vi "Main.vi"() -> ()   [LabVIEW 2020] (continued)
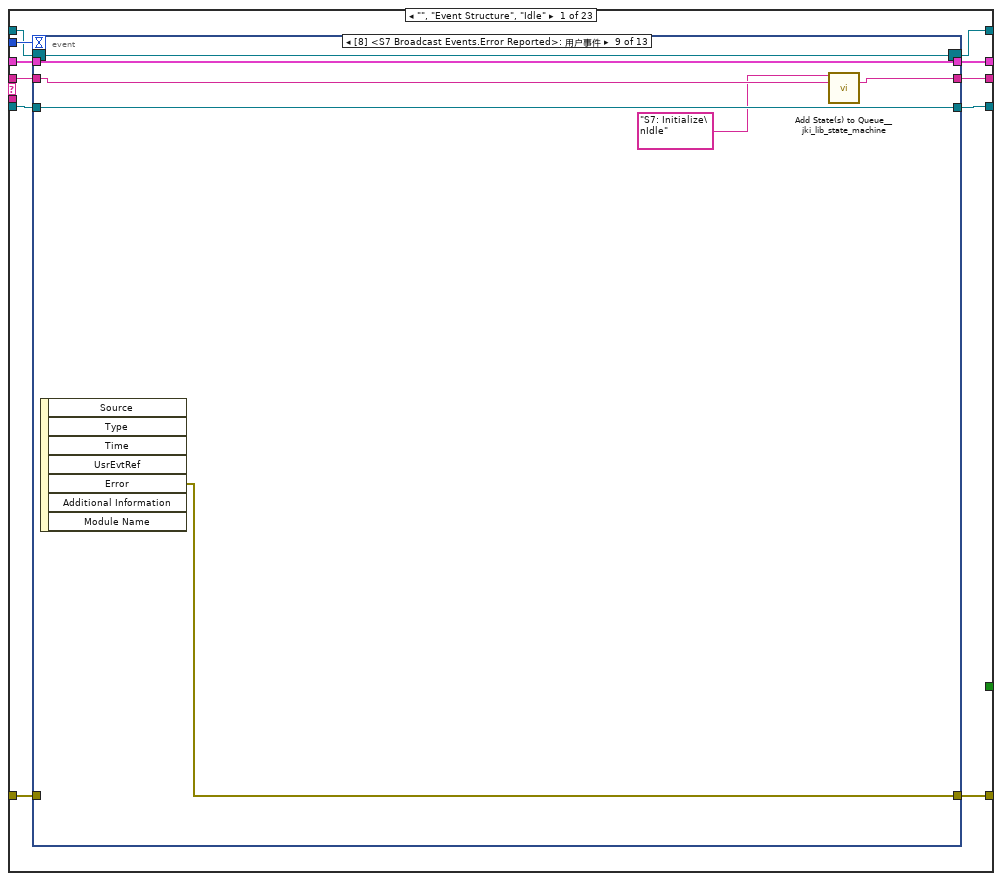
[diagram p2: hidden frame]
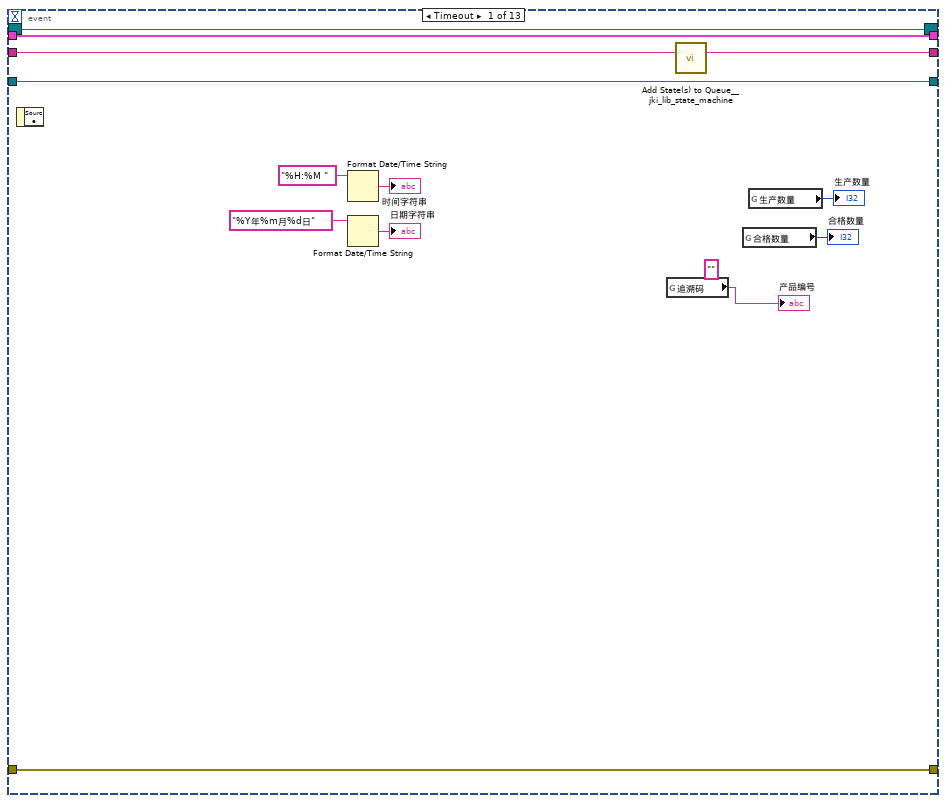
[diagram p3: hidden frame]
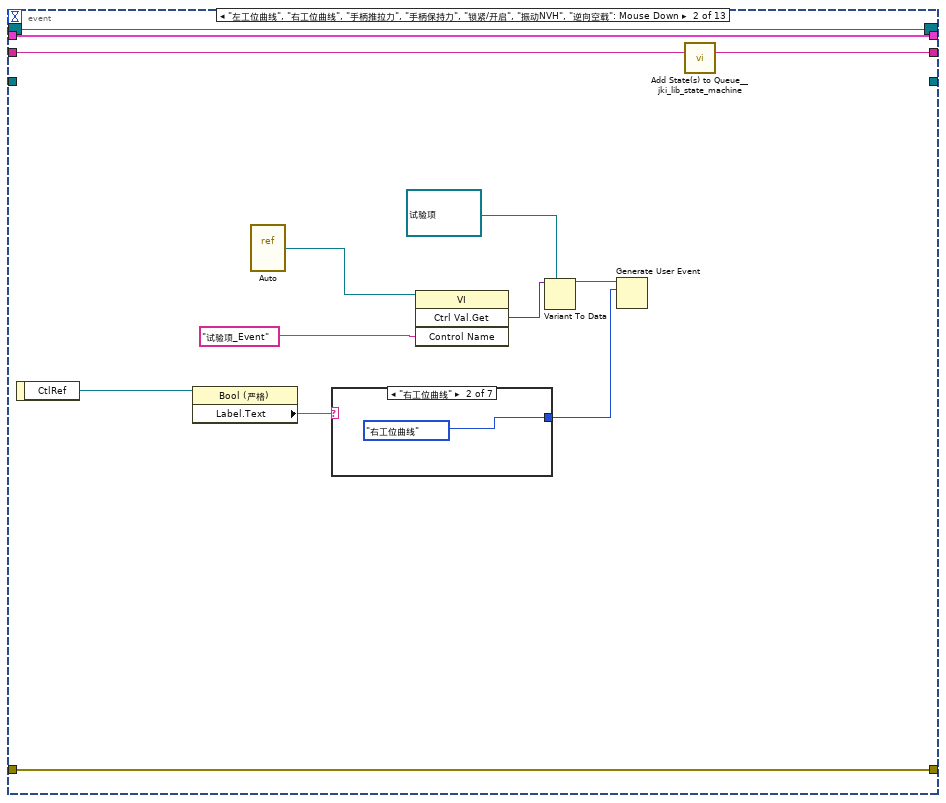
[diagram p4: hidden frame]
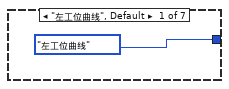
[diagram p5: hidden frame]
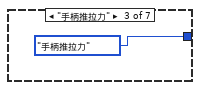
[diagram p6: hidden frame]
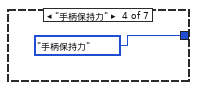
[diagram p7: hidden frame]
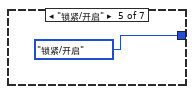
[diagram p8: hidden frame]
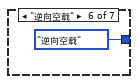
[diagram p9: hidden frame]
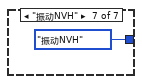
[diagram p10: hidden frame]
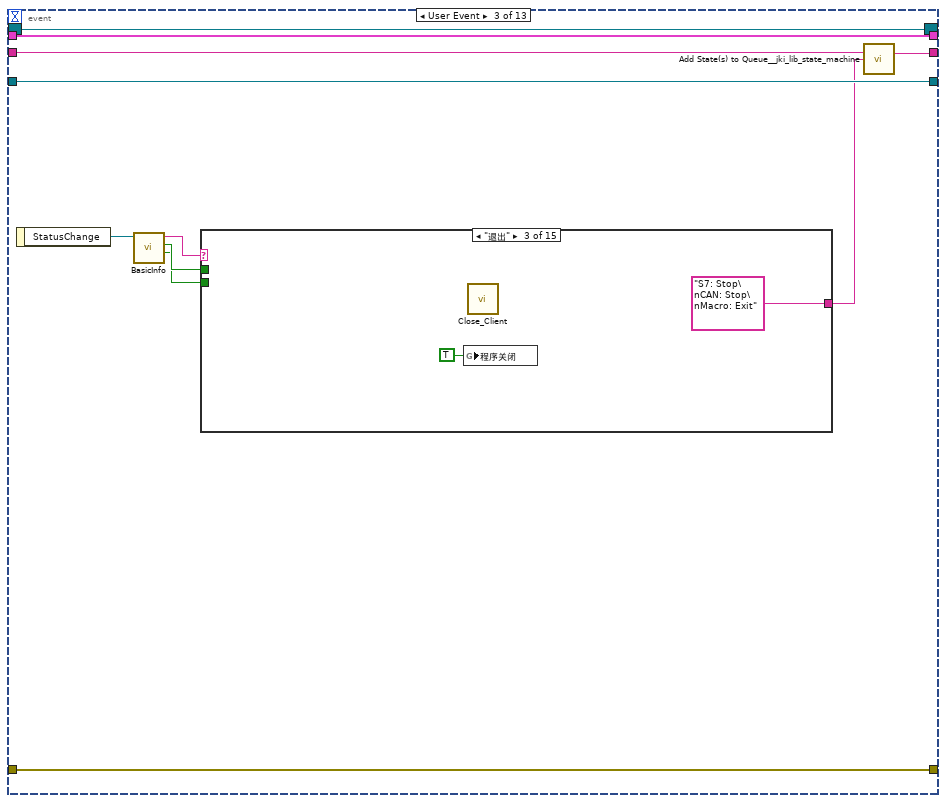
[diagram p11: hidden frame]
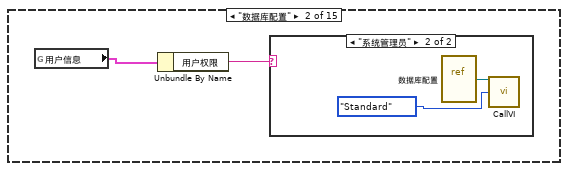
[diagram p13: hidden frame]
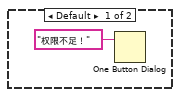
[diagram p14: hidden frame]
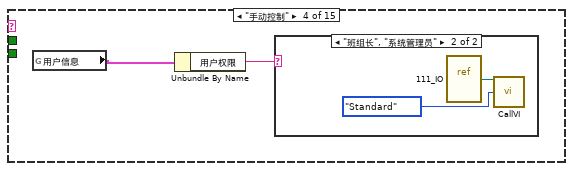
[diagram p15: hidden frame]
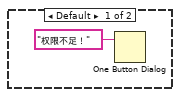
[diagram p16: hidden frame]
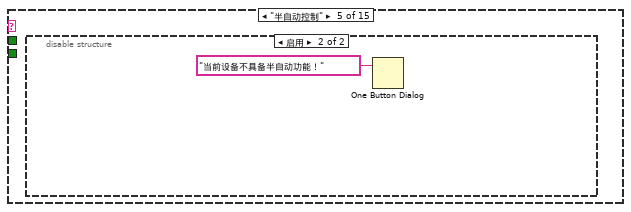
[diagram p17: hidden frame]
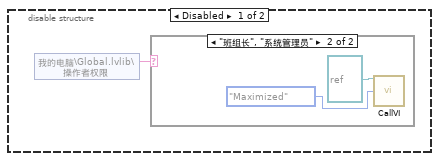
[diagram p18: hidden frame]
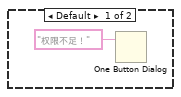
[diagram p19: hidden frame]
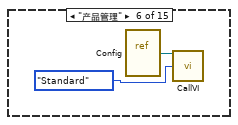
[diagram p20: hidden frame]
            n115 = call "CallVI.vi"("VI引用"=w195, "状态"=T6."Standard") -> ()  [unwired: 11 in, 3 out]
            n116 = call <vilib>:"Add State(s) to Queue__jki_lib_state_machine.vi"("State(s) in (\"\")"=w197) -> ("States Out"=w198:string)  [unwired: 14 in]
          }
          event Panel Close? {
            n117 = event-data() -> ()  [unwired: 1 in, 1 out]
            n118 = global write "Global.vi" "程序关闭"(TRUE ("程序关闭")) -> ()
            n119 = call <vilib>:"Add State(s) to Queue__jki_lib_state_machine.vi"("State(s) in Front (\"\")"="S7: Stop\nMacro: Exit", "State(s) in (\"\")"=w207) -> ("States Out"=w206:string)  [unwired: 13 in]
            n120 = event-data("Discard?"=TRUE) -> ()  [unwired: 1 in, 1 out]
          }
          event "产品更换": Value Change {
            n121 = event-data() -> ("NewVal"=w212:refnum<vi>)  [unwired: 1 in, 5 out]
            n122 = stacked-sequence {
              tunnel: w212 -> [w222 _]
              tunnel: [_ "Idle" ("State(s) in Front (\"\")")] -> w208
              frame #0 {
                n123 = disable-structure shown="禁用" {
                  disable-tunnel: w222 -> [w224 _]
                  frame Disabled {
                    n124 = control-ref of="子面板"() -> (w223:refnum<vi>)
                    n125 = call "Call_SubPanal.vi"("VI引用句柄"=w224, "SubPnl引用句柄"=w223) -> ()  [unwired: 9 in, 1 out]
                  }
                  frame Enabled {
                  }
                }
                n126 = vi-ref "Auto.vi"() -> (w216:refnum<vi>)
                n127 = global read "Global.vi" "产品型号"() -> (w215:string)
                n128 = invoke class="VI" method="Ctrl Val.Get"(reference=w216, "Control Name"="标尺_Event" ("控件名")) -> ("Get Control Value Variant"=w221:variant)  [unwired: 2 in, 3 out]
                n129 = Variant To Data(type=refnum<user-event> refnum ("标尺_Event"), Variant=w221) -> (data=w218:refnum<user-event>, error out=w217:errorcluster)  [unwired: 1 in]
                n130 = Generate User Event(user event=w218, event data cluster=w215, error in=w217) -> ()  [unwired: 1 in, 2 out]
                n131 = local write "产品型号"(w215) -> ()
              }
              frame #1 {
                n132 = control-ref of="锁紧/开启"() -> (w226:refnum<vi>)
                n133 = control-ref of="手柄保持力"() -> (w227:refnum<vi>)
                n134 = control-ref of="左工位曲线"() -> (w228:refnum<vi>)
                n135 = control-ref of="右工位曲线"() -> (w229:refnum<vi>)
                n136 = control-ref of="手柄推拉力"() -> (w230:refnum<vi>)
                n137 = global read "Global.vi" "试验项目"() -> (w233:bool[])
                n138 = Build Array(w228, w229, w230, w227, w226) -> (w232:refnum<vi>[])
                n139 = for {
                  tunnel: w232 -> [w237] mode=indexing
                  tunnel: w233 -> [w238] mode=indexing
                  shift-right: [w234] -> _
                  shift-left: 2000 -> [w235]
                  i -> [w236]
                  n140 = case shown="真" w238 {
                    tunnel: w237 -> [w239 w247]
                    tunnel: w236 -> [_ _]
                    tunnel: w235 -> [w241 w244]
                    tunnel: [w241 w242] -> w234
                    frame False {
                      n141 = property class="Bool (严格)"(reference=w239, "Top"=2000) -> ()  [unwired: 1 in, 2 out]
                    }
                    frame True {
                      n142 = Add(x=w244, y=180) -> (x+y=w242:i32)
                      n143 = Bundle(w242, 1230) -> (w245:cluster{i32, i32})  [unwired: 1 in]
                      n144 = property class="Bool (严格)"(reference=w247, "Position"=w245) -> ()  [unwired: 1 in, 2 out]
                    }
                  }
                }
              }
            }
            n145 = call <vilib>:"Add State(s) to Queue__jki_lib_state_machine.vi"("State(s) in Front (\"\")"=w208, "State(s) in (\"\")"=w210) -> ("States Out"=w209:string)  [unwired: 13 in]
          }
          event "Andon": Value Change {
            n146 = event-data() -> ("NewVal"=w252:enum32{"未选择", "缺料报警", "质量报警", "故障报警"})  [unwired: 1 in]
            n147 = case shown="\"未选择\", 默认" w252 {
              tunnel: [enum16{"设备离线", "设备正常", "设备缺料", "设备故障", "质量报警"}."设备正常" ("设备状态") enum16{"设备离线", "设备正常", "设备缺料", "设备故障", "质量报警"}."设备缺料" ("设备状态") enum16{"设备离线", "设备正常", "设备缺料", "设备故障", "质量报警"}."质量报警" ("设备状态") enum16{"设备离线", "设备正常", "设备缺料", "设备故障", "质量报警"}."设备故障" ("设备状态")] -> w250
              frame "未选择", Default {
              }
              frame "缺料报警" {
              }
              frame "质量报警" {
              }
              frame "故障报警" {
              }
            }
            n148 = local read "userName"() -> (w249:string)
            n149 = Bundle By Name(cluster=T7 {"设备名称"="调节机构检测", "操作人员"="", "设备状态"=enum."设备离线", "附加信息"=""} ("设备信息"), "操作人员"=w249, "设备状态"=w250) -> (w248:T7)
            n150 = call "Change_Client.vi"("设备信息"=w248) -> ()  [unwired: 10 in, 1 out]
          }
        }
      }
      frame "---------- Core ----------" {
        n151 = call <vilib>:"Add State(s) to Queue__jki_lib_state_machine.vi"("State(s) in (\"\")"=w266) -> ("States Out"=w265:string)  [unwired: 14 in]
      }
      frame Default {
        w278 = 42 items=["No error", "Argument error", "Memory is full", "Out of zone", "End of file", "File already open", "Generic file I/O error", "File not found", "File permission error", "Disk is full", "Duplicate path", "Too many files open", "System feature not enabled", "Resource file not found", "Cannot add resource", "Resource not found", "Image not found", "Image memory error", "Pen does not exist", "Config type invalid", "Config token not found", "Config parse error", "Config memory error", "Bad external code format", "Bad external code offset", "External code not present", "Null window", "Destroy window error", "Null menu", "Print aborted", "Bad print record", "Print driver error", "Windows error during printing", "Memory error during printing", "Print dialog error", "Generic print error", "Invalid device refnum", "Device not found", "Device parameter error", "Device unit error", "Cannot open device", "Device call aborted", "Generic error", "Cancelled by user", "Object ID too low", "Object ID too high", "Object not in heap", "Unknown heap", "Unknown object (invalid DefProc)", "Unknown object (DefProc not in table)", "Message out of range", "Invalid (null) method", "Unknown message", "Manager call not supported", "Bad address", "Network operation in progress", "Network operation timed out", "Connection is busy", "Network attribute not supported", "Network error", "Address in use", "System out of memory", "Connection aborted", "Connection refused", "Not connected", "Already connected", "Connection closed", "Initialization error (interapplication manager)", "Bad occurrence", "Wait on unbound occurrence handler", "Occurrence queue overflow", "Datalog type conflict", "Unused", "Unrecognized type (interapplication manager)", "Memory corrupt", "Failed to make temporary DLL", "Old CIN version", "Drag socket not found", "Failed to load drop-object", "Failed to register OLE object", "Failed to release OLE object", "Format specifier type mismatch", "Unknown format specifier", "Too few format specifiers", "Too many format specifiers", "Scan failed", "Newer CIN version", "Error converting to variant", "Runtime menu error", "Password tampered", "Variant attribute not found", "Incompatible variant data type", "Event data is not available", "Event Store is not present", "Occurrence is not found", "Event Queue is not created", "Event info is not available", "Refnum passed is NULL", "Error retrieving Class GUID", "Error retrieving CoClass GUID", "Error retrieving TypeLib GUID.", "Bad built application magic bytes.", "Specific driver is different from the specific driver associated with the Logical Name.", "There is no session opened to the class driver.", "Max Error", "MAX - Error with config objects", "MAX - Error loading configuration", "MAX - Group not supported"]
        # "Current State"
        n152 = Format Into String(format string="Software Exception: Unhandled State \"%s\"." ("message"), error in=w274, w269) -> (resulting string=w277:string, error out=w276:errorcluster)  [unwired: 1 in]
        n153 = call <vilib>:"Error Cluster From Error Code.vi"("show call chain? (False)"=TRUE, "error in (no error)"=w276, "error message (\"\")"=w277, "error code (0)"=w278) -> ("error out"=w275:errorcluster)  [unwired: 5 in]
        n154 = call <vilib>:"Add State(s) to Queue__jki_lib_state_machine.vi"("State(s) in (\"\")"=w273) -> ("States Out"=w272:string)  [unwired: 14 in]
      }
      frame "Initialize Core Data" {
        # "originally closed?"
        # "exe?"
        n155 = property class="VI"() -> ("Front Panel.Open"=w289:bool)  [unwired: 2 in, 2 out]
        n156 = property class="App"() -> ("App.Kind"=w288:T8)  [unwired: 2 in, 2 out]
        n157 = control-ref of="Current VI Reference"() -> (w282:refnum<vi>)
        n158 = Not(x=w289) -> (.not. x?=w286:bool)
        n159 = Equal?(x=w288, y=T8."Run Time System" ("Application:Kind")) -> (x = y?=w285:bool)
        n160 = Or(x=w286, y=w285) -> (x .or. y?=w283:bool)
        n161 = Bundle By Name(cluster=w284, "Core.Current VI Reference"=w282, "Core.Close Panel on Exit?"=w283) -> (w291:T10)
        n162 = call <vilib>:"Add State(s) to Queue__jki_lib_state_machine.vi"("State(s) in (\"\")"=w293) -> ("States Out"=w292:string)  [unwired: 14 in]
      }
      frame "Error Handler" {
        n163 = call <vilib>:"General Error Handler.vi"("error in (no error)"=w297) -> ()  [unwired: 10 in, 5 out]
        n164 = call <vilib>:"Add State(s) to Queue__jki_lib_state_machine.vi"("State(s) in Front (\"\")"="/* Post Error States", "State(s) in (\"\")"=w301) -> ("States Out"=w300:string)  [unwired: 13 in]
      }
      frame "Exit" {
        n165 = call <vilib>:"Add State(s) to Queue__jki_lib_state_machine.vi"("State(s) in (\"\")"=w308) -> ("States Out"=w307:string)  [unwired: 14 in]
        n166 = Quit LabVIEW() -> ()  [unwired: 1 in]
      }
      frame "--------- Library --------" {
        n167 = call <vilib>:"Add State(s) to Queue__jki_lib_state_machine.vi"("State(s) in (\"\")"=w314) -> ("States Out"=w313:string)  [unwired: 14 in]
      }
      frame "S7: Initialize" {
        n168 = property on="PLC" class="Bool (严格)"("Val(Sgnl)"=FALSE ("值(信号)")) -> ()  [unwired: 2 in, 2 out]
      }
      frame "S7: Stop" {
        n169 = call "Stop Module.vi"("error in (no error)"=w322) -> ("error out"=w321:errorcluster)  [unwired: 10 in]
        n170 = call <vilib>:"Add State(s) to Queue__jki_lib_state_machine.vi"("State(s) in (\"\")"=w324) -> ("States Out"=w325:string)  [unwired: 14 in]
      }
      frame "CAN: Start" {
        n171 = call <vilib>:"Add State(s) to Queue__jki_lib_state_machine.vi"("State(s) in (\"\")"=w330) -> ("States Out"=w331:string)  [unwired: 14 in]
      }
      frame "CAN: Stop" {
        n172 = call <vilib>:"Add State(s) to Queue__jki_lib_state_machine.vi"("State(s) in (\"\")"=w336) -> ("States Out"=w337:string)  [unwired: 14 in]
      }
      frame "---------- Data ----------" {
        n173 = call <vilib>:"Add State(s) to Queue__jki_lib_state_machine.vi"("State(s) in (\"\")"=w345) -> ("States Out"=w344:string)  [unwired: 14 in]
      }
      frame "Data: Initialize" {
        w350 = T11 {"Current VI Reference"=refnum, "Close Panel on Exit?"=FALSE}  # Core
        w352 = TRUE  # Your Boolean data
        w351 = ""  # Your string data
        n174 = call "Fit VI window to Content__ogtk.vi"("border spacing (2 px)"=0) -> ()  [unwired: 5 in, 2 out]
        n175 = global write "Global.vi" "程序关闭"(FALSE ("程序关闭")) -> ()
        n176 = Bundle("Core"=w350, "Your Boolean data"=w352, "Your string data"=w351) -> (w354:T10)  [unwired: 1 in]
        n177 = call <vilib>:"Add State(s) to Queue__jki_lib_state_machine.vi"("State(s) in (\"\")"=w356) -> ("States Out"=w355:string)  [unwired: 14 in]
      }
      frame "Data: Cleanup" {
        n178 = Unbundle By Name(w359) -> ("Core.Current VI Reference"=w362:refnum<vi>)
        n179 = Close Reference(reference=w362, error in (no error)=w361) -> (error out=w360:errorcluster)
        n180 = call <vilib>:"Add State(s) to Queue__jki_lib_state_machine.vi"("State(s) in (\"\")"=w364) -> ("States Out"=w363:string)  [unwired: 14 in]
      }
      frame "---------- UI ----------" {
        # "Do not put any code in this frame.\n(It is a separator no-op. You can make a copy of this frame to create a new UI frame)"
        n181 = call <vilib>:"Add State(s) to Queue__jki_lib_state_machine.vi"("State(s) in (\"\")"=w370) -> ("States Out"=w369:string)  [unwired: 14 in]
      }
      frame "UI: Initialize" {
        n182 = disable-structure shown="启用" {
          disable-tunnel: [w384 _] -> w374
          disable-tunnel: w371 -> [w382 _]
          frame Enabled {
            n183 = vi-ref "Auto.vi"() -> (w383:refnum<vi>)
            n184 = property class="VI"(reference=w383) -> (reference out=w381:refnum<vi>, "FP.State"=w380:T6)  [unwired: 1 in, 1 out]
            n185 = case shown="\"Standard\", 默认" w380 {
              tunnel: w382 -> [w390 w392]
              tunnel: w381 -> [w391 w393]
              tunnel: [w389 w393] -> w378
              tunnel: [w388 w392] -> w379
              frame "Standard", Default {
                n186 = invoke class="VI" method="FP.Close"(reference=w391, error in=w390) -> (reference out=w389:refnum<vi>, error out=w388:errorcluster)  [unwired: 1 in, 1 out]
              }
              frame "Invalid", "Closed" {
              }
            }
            n187 = invoke on="子面板" class="SubPnl" method="Insert VI"(error in=w379, "VI Ref"=w378) -> (error out=w387:errorcluster)  [unwired: 2 in, 3 out]
            n188 = invoke class="VI" method="Run VI"(reference=w378, error in=w387, "Wait until done"=FALSE ("结束前等待"), "Auto Dispose Ref"=TRUE ("自动销毁引用")) -> (error out=w384:errorcluster)  [unwired: 1 in, 4 out]
          }
          frame Disabled {
            n189 = vi-ref "Auto.vi"() -> (w395:refnum<vi>)
            n190 = call "CallVI.vi"("VI引用"=w395, "状态"=T6."Maximized") -> ()  [unwired: 11 in, 3 out]
          }
        }
        n191 = call <vilib>:"Add State(s) to Queue__jki_lib_state_machine.vi"("State(s) in (\"\")"=w377) -> ("States Out"=w376:string)  [unwired: 14 in]
      }
      frame "UI: Init" {
        n192 = stacked-sequence {
          tunnel: w397 -> [_ _ _ _ _]
          frame #0 {
            n193 = property on="上学状态" class="Str"("Text.BGColor"=u32 16777216 ("文本.文本颜色:背景色")) -> ()  [unwired: 2 in, 2 out]
          }
          frame #1 {
            n194 = global write "Global.vi" "程序关闭"(FALSE ("程序关闭")) -> ()
            n195 = control-ref of="右工位曲线"() -> (w404:refnum<vi>)
            n196 = control-ref of="左工位曲线"() -> (w403:refnum<vi>)
            n197 = global write "A131258.vi" "LED-左工位"(w403) -> ()
            n198 = global write "A131258.vi" "LED-右工位"(w404) -> ()
            n199 = control-ref of="上学状态"() -> (w405:refnum<vi>)
            n200 = global write "Global.vi" "上序状态"(w405) -> ()
          }
          frame #2 {
            w416 = 0
            n201 = global read "Global.vi" "上序状态"() -> (w413:refnum<vi>)
            n202 = shared-variable "我的电脑\\Global.lvlib\\工位追溯码"("   " ("工位追溯码")) -> ()  [unwired: 1 in, 1 out]
            n203 = global write "Global.vi" "生产数量"(w416) -> ()
            n204 = global write "Global.vi" "合格数量"(w416) -> ()
            n205 = global read "Global1.vi" "用户信息"() -> (w412:T9)
            n206 = property class="Str"(reference=w413, "Value"="" ("值"), "Text.BGColor"=u32 16777216 ("文本.文本颜色:背景色")) -> ()  [unwired: 1 in, 2 out]
            n207 = global read "Global1.vi" "联机模式"() -> (w409:enum16{"单机", "追溯"})
            n208 = Unbundle By Name(w412) -> ("用户名"=→"userName":string, "用户权限"=→"userStatus":string)
            n209 = case shown="\"追溯\"" w409 {
              tunnel: ["联网" ("connectionMode") "单机" ("connectionMode")] -> w417
              frame "追溯" {
              }
              frame "单机", Default {
              }
            }
            "connectionMode" <- w417
            "产品型号" <- "" ("产品型号")
          }
          frame #3 {
            n210 = control-ref of="表格控件"() -> (w421:refnum<vi>)
            n211 = control-ref of="提示信息"() -> (w422:refnum<vi>)
            n212 = control-ref of="自动"() -> (w423:refnum<vi>)
            n213 = control-ref of="错误"() -> (w424:refnum<vi>)
            n214 = control-ref of="产品更换"() -> (w420:refnum<vi>)
            n215 = global write "Global.vi" "提示信息"(w422) -> ()
            n216 = global write "Global.vi" "程序自动"(w423) -> ()
            n217 = global write "Global.vi" "报警图标"(w424) -> ()
            n218 = global write "Global.vi" "Result"(w421) -> ()
            n219 = global write "Global.vi" "更换产品"(w420) -> ()
          }
          frame #4 {
            w425 = -2
            n220 = global read "Global.vi" "Result"() -> (w428:refnum<vi>)
            n221 = property class="Tbl"(reference=w428, "Row Headers[]"=string[] [], "Value"=string[][] []) -> ()  [unwired: 1 in, 2 out]
            n222 = Bundle(w425, w425) -> (w426:cluster{i32, i32})  [unwired: 1 in]
            n223 = property class="Tbl"(reference=w428, "Active Cell"=w426, "Cell BG Color"=u32 16777216 ("活动单元格:单元格背景色")) -> ()  [unwired: 1 in, 2 out]
            n224 = call "Start_Client.vi"() -> ()  [unwired: 12 in]
          }
        }
        n225 = call <vilib>:"Add State(s) to Queue__jki_lib_state_machine.vi"("State(s) in (\"\")"=w401) -> ("States Out"=w400:string)  [unwired: 14 in]
      }
      frame "UI: Config" {
        n226 = vi-ref "Config.vi"() -> (w433:refnum<vi>)
        n227 = call "CallVI.vi"("VI引用"=w433, "状态"=T6."Standard") -> ()  [unwired: 11 in, 3 out]
        n228 = call <vilib>:"Add State(s) to Queue__jki_lib_state_machine.vi"("State(s) in (\"\")"=w438) -> ("States Out"=w437:string)  [unwired: 14 in]
      }
      frame "UI: Cursor Set" {
        # "Argument"
        n229 = case shown="\"Idle\", 默认" w441 {
          tunnel: w443 -> [w448 w450]
          tunnel: [w447 w449] -> w442
          frame "Idle", Default {
            n230 = call <vilib>:"Unset Busy.vi"("error in (no error)"=w448) -> ("error out"=w447:errorcluster)  [unwired: 10 in]
          }
          frame "Busy" {
            n231 = call <vilib>:"Set Busy.vi"("error in (no error)"=w450) -> ("error out"=w449:errorcluster)  [unwired: 9 in, 1 out]
          }
        }
        n232 = call <vilib>:"Add State(s) to Queue__jki_lib_state_machine.vi"("State(s) in (\"\")"=w446) -> ("States Out"=w445:string)  [unwired: 14 in]
      }
      frame "UI: Front Panel State" {
        # "Argument"
        n233 = Unbundle By Name(w455) -> ("Core.Current VI Reference"=w454:refnum<vi>)
        n234 = case shown="\"Close\"" w453 {
          tunnel: w457 -> [w463 w476]
          tunnel: [w465 w477] -> w456
          tunnel: w454 -> [w464 w474]
          frame "Open", Default {
            n235 = property class="VI"(reference=w464, error in=w463) -> (reference out=w461:refnum<vi>, error out=w462:errorcluster, "Front Panel.Open"=w460:bool)
            n236 = case shown="假" w460 {
              tunnel: [w468 w471] -> w465
              tunnel: w462 -> [w467 w471]
              tunnel: w461 -> [w466 _]
              frame False {
                n237 = invoke class="VI" method="FP.Open"(reference=w466, error in=w467, "Activate"=TRUE, "State"=T6."Standard") -> (error out=w468:errorcluster)  [unwired: 1 in, 4 out]
              }
              frame True {
              }
            }
          }
          frame "Close" {
            n238 = property class="VI"(reference=w474, error in=w476) -> (reference out=w473:refnum<vi>, error out=w475:errorcluster, "Front Panel.Open"=w472:bool)
            n239 = case shown="真" w472 {
              tunnel: [w478 w481] -> w477
              tunnel: w475 -> [w478 w480]
              tunnel: w473 -> [_ w479]
              frame False {
              }
              frame True {
                n240 = invoke class="VI" method="FP.Close"(reference=w479, error in=w480) -> (error out=w481:errorcluster)  [unwired: 1 in, 2 out]
              }
            }
          }
        }
        n241 = call <vilib>:"Add State(s) to Queue__jki_lib_state_machine.vi"("State(s) in (\"\")"=w459) -> ("States Out"=w458:string)  [unwired: 14 in]
      }
      frame "---------- Macro ----------" {
        n242 = call <vilib>:"Add State(s) to Queue__jki_lib_state_machine.vi"("State(s) in (\"\")"=w487) -> ("States Out"=w486:string)  [unwired: 14 in]
      }
      frame "Macro: Initialize" {
        n243 = call <vilib>:"Add State(s) to Queue__jki_lib_state_machine.vi"("State(s) in Front (\"\")"="Data: Initialize\nInitialize Core Data\nS7: Initialize\nIdle\nUI: Init\nUI: Front Panel State >> Open\nUI: Initialize\nUI: Config", "State(s) in (\"\")"=w494) -> ("States Out"=w493:string)  [unwired: 13 in]
      }
      frame "Macro: Exit" {
        n244 = Unbundle By Name(w503) -> ("Core.Close Panel on Exit?"=w502:bool)
        n245 = Select(t="UI: Front Panel State >> Close", s=w502, f="") -> (s? t:f=w499:string)
        n246 = call <vilib>:"Add State(s) to Queue__jki_lib_state_machine.vi"("State(s) in (\"\")"=w499, "State(s) at Back (\"\")"="Data: Cleanup\nExit") -> ("States Out"=w497:string)  [unwired: 13 in]
        n247 = call <vilib>:"Add State(s) to Queue__jki_lib_state_machine.vi"("State(s) in Front (\"\")"=w497, "State(s) in (\"\")"=w506) -> ("States Out"=w505:string)  [unwired: 13 in]
      }
    }
  }
  n248 = call-dynamic "Cleanup.vi"("MenuStrip in"=w6) -> ()  [unwired: 10 in, 1 out]
